vi "UHR-Fleezers Control (host) - 10.3.vi"() -> ()   [LabVIEW 2010] (continued)
            n263 = local write "Overflow (data lost)"(FALSE ("Overflow (data lost)")) -> ()
          }
        }
        n264 = case shown="False" w2065 {
          selector: w2065 -> [_ w2081]
          tunnel: w2064 -> [w2080 _]
          tunnel: [w2080 w2081] -> w2063
          frame False {
            n265 = property on="2D or 1D Scan" class="Bool (strict)"("Val(Sgnl)"=w2080) -> ()  [unwired: 2 in, 2 out]
            n266 = property on="Confocal Image" class="Bool (strict)"("Value"=FALSE ("Start Confocal Map")) -> ()  [unwired: 2 in, 2 out]
          }
          frame True {
          }
        }
        n267 = local write "MCL Scanning"(w2070) -> ()
        n268 = local read "AO1"() -> (w2067:dbl)
        n269 = local read "AO2"() -> (w2066:dbl)
        n270 = case shown="True" "Center Scan" {
          tunnel: w2075 -> [w2088 w2200]
          tunnel: w2074 -> [w2087 w2199]
          tunnel: [w2086 w2198] -> w2072
          tunnel: [w2085 w2197] -> w2071
          tunnel: [w2083 w2184] -> w2069
          tunnel: [w2082 w2183] -> w2068
          tunnel: w2067 -> [w2083 w2189]
          tunnel: w2066 -> [w2082 w2192]
          tunnel: w2063 -> [_ _]
          frame False {
            w2084 = TRUE ("AI to FIFO")
            n271 = xnode "Read/Write Control"("FPGA VI Reference In"=w2088, "error in"=w2087, "AI to FIFO"=w2084, "APD to FIFO"=w2084, "Start scan (MCL)"=w2084) -> ("FPGA VI Reference Out"=w2086:T19, "error out"=w2085:errorcluster)
          }
          frame True {
            w2196 = TRUE ("AI to FIFO")
            n272 = local read "Scan steps (MCL)"() -> (w2175:u64)
            n273 = local read "Scan lines (y)"() -> (w2171:u64)
            n274 = local read "Fast Scan Dir"() -> (w2182:bool)
            n275 = local read "Actual MCL Inc (V)"() -> (w2172:dbl)
            n276 = Decrement(x=w2171) -> (x-1=w2170:u64)
            n277 = Decrement(x=w2175) -> (x-1=w2174:u64)
            n278 = Multiply(x=w2172, y=w2170) -> (x*y=w2169:dbl)
            n279 = Divide(x=w2169, y=2.0) -> (x/y=w2179:dbl)
            n280 = Multiply(x=w2172, y=w2174) -> (x*y=w2173:dbl)
            n281 = Divide(x=w2173, y=2.0) -> (x/y=w2178:dbl)
            n282 = Select(t=w2178, s=w2182, f=w2179) -> (s? t:f=w2177:dbl)
            n283 = Select(t=w2179, s=w2182, f=w2178) -> (s? t:f=w2181:dbl)
            n284 = Subtract(x=w2189, y=w2181) -> (x-y=w2180:dbl)
            n285 = Subtract(x=w2192, y=w2177) -> (x-y=w2176:dbl)
            n286 = local read "2D or 1D Scan"() -> (w2194:bool)
            n287 = Not(x=w2182) -> (.not. x?=w2188:bool)
            n288 = Not(x=w2194) -> (.not. x?=w2190:bool)
            n289 = And(x=w2182, y=w2190) -> (x .and. y?=w2191:bool)
            n290 = And(x=w2190, y=w2188) -> (x .and. y?=w2193:bool)
            n291 = Select(t=w2192, s=w2193, f=w2176) -> (s? t:f=w2183:dbl)
            n292 = Select(t=w2189, s=w2191, f=w2180) -> (s? t:f=w2184:dbl)
            n293 = call "Volt to I16.vi"("Voltage In"=w2184) -> ("I16 Voltage Out"=w2187:i16)
            n294 = call "Volt to I16.vi"("Voltage In"=w2183) -> ("I16 Voltage Out"=w2186:i16)
            n295 = xnode "Read/Write Control"("FPGA VI Reference In"=w2200, "error in"=w2199, "AI to FIFO"=w2196, "APD to FIFO"=w2196, "Start scan (MCL)"=w2196, "AO1"=w2187, "AO2"=w2186) -> ("FPGA VI Reference Out"=w2198:T19, "error out"=w2197:errorcluster)
          }
        }
        "Initial Y" <- w2069
        "Initial X" <- w2068
        "wait to reset values" <- w2070
      }
    }
    n296 = local read "Trap Pos Elements/DMA read"() -> (w1019:u32)
    n297 = local read "Trap AI Elements/DMA read"() -> (w1104:u32)
    n298 = local read "APD Elements/DMA read"() -> (w1064:u32)
    n299 = xnode "Get APD Data"("FPGA VI Reference In"=w1023, "error in"=w1022, "Number of Elements"=w1064, "Timeout (ms)"=-1) -> ("Data"=w1063:u32[], "Elements Remaining"=→"APD FIFO Elements Remaining":u32)  [unwired: 2 out]
    n300 = xnode "Invoke Method"("FPGA VI Reference In"=w1023, "error in"=w1022, "Number of Elements"=w1019, "Timeout (ms)"=-1) -> ("Data"=w982:u16[], "Elements Remaining"=→"Trap Pos FIFO El Remaining":u32)  [unwired: 2 out]
    n301 = xnode "Get Trap Data"("FPGA VI Reference In"=w1023, "error in"=w1022, "Number of Elements"=w1104, "Timeout (ms)"=-1 ("Timeout")) -> ("FPGA VI Reference Out"=w1093:T19, "error out"=w1092:errorcluster, "Data"=w983:i16[], "Elements Remaining"=w1239:u32)
    "FIFO El. Rem." <- w1239
    n302 = local read "Trap AI FIFO Depth"() -> (w1241:u32)
    n303 = Subtract(x=w1241, y=w1104) -> (x-y=w1240:u32)
    n304 = Decimate 1D Array(w982) -> (w979:u16[], w981:u16[], w980:u16[])
    n305 = Divide(x=w1239, y=w1240) -> (x/y=w1238:dbl)
    "Buffer Status" <- w1238
    n306 = To Unsigned Long Integer(number=w979) -> (unsigned 32bit integer=w978:u32[])
    n307 = Join Numbers(hi=w981, lo=w980) -> ((hi.lo)=w977:u32[])
    n308 = Equal?(x=w1238, y=1.0) -> (x = y?=w1236:bool)
    n309 = Join Numbers(hi=w978, lo=w977) -> ((hi.lo)=w971:u64[])
    n310 = call "IR AOM word to freq - vec.vi"("Frequency Word In (double vec)"=w971) -> ("Frequency Out"=w1018:dbl[])
    n311 = case "Alert buffer overflow" shown="True" w1236 {
      frame False {
      }
      frame True {
        n312 = call <vilib>:"Beep.vi"() -> ()  [unwired: 3 in, 9 out]
        "Overflow (data lost)" <- TRUE ("Overflow (data lost)")
      }
    }
    n313 = Decimate 1D Array(w1018) -> (w1017:dbl[], w1016:dbl[])
    n314 = Build Array(w1017, w1016) -> (w1015:dbl[][])
    n315 = local read "Trap Sets"() -> (w1103:u32)
    n316 = case "Deinterlace trap data, average down PSD" shown="1, Default" w1103 {
      tunnel: w983 -> [w2357 w2422]
      tunnel: [w2354 w2419] -> w1096
      tunnel: [w2357 w2421] -> w974
      tunnel: "Detector Type" -> [w2356 w2417]
      tunnel: [w2355 w2420] -> w1095
      tunnel: [w2353 w2418] -> w1211
      frame 1, Default {
        n317 = Divide(x=w2357, y=3276.7) -> (x/y=w2358:dbl[])
        n318 = Decimate 1D Array(w2358) -> (w2367:dbl[], w2366:dbl[], w2365:dbl[], w2364:dbl[], w2363:dbl[], w2362:dbl[], w2361:dbl[], w2360:dbl[])
        n319 = case shown="\"IR-QPD + PSD + FB-QPD position\"" w2356 {
          tunnel: w2367 -> [w2391 w2416]
          tunnel: w2366 -> [w2390 w2415]
          tunnel: w2365 -> [w2375 w2393]
          tunnel: w2364 -> [w2376 w2403]
          tunnel: w2363 -> [w2389 w2414]
          tunnel: w2362 -> [w2388 w2413]
          tunnel: w2361 -> [w2372 w2394]
          tunnel: w2360 -> [w2371 w2392]
          tunnel: [w2370 w2400] -> w2355
          tunnel: [w2369 w2399] -> w2354
          tunnel: [w2368 w2398] -> w2353
          frame "IR-QPD + PSD + FB-QPD", Default {
            w2368 = 0  # Channel pattern
            n320 = Divide(x=w2391, y=w2376) -> (x/y=w2378:dbl[])
            n321 = Divide(x=w2390, y=w2376) -> (x/y=w2377:dbl[])
            n322 = Divide(x=w2389, y=w2372) -> (x/y=w2374:dbl[])
            n323 = Divide(x=w2388, y=w2371) -> (x/y=w2373:dbl[])
            n324 = Build Array(w2378, w2377, w2376, w2375, w2374, w2373, w2372, w2371) -> (w2369:dbl[][])
            n325 = Bundle("T1 Y", "T1 X", "T1 Sum", "FB Sum", "PSD Y", "PSD X", "PSD Y Sum", "PSD X Sum") -> (w2387:T35)  [unwired: 1 out]
            n326 = Cluster To Array(cluster=w2387) -> (array=w2370:string[])
          }
          frame "IR-QPD + PSD + FB-QPD position" {
            w2398 = 3  # Channel pattern
            n327 = Negate(x=w2394) -> (-x=w2395:dbl[])
            n328 = Divide(x=w2416, y=w2403) -> (x/y=w2405:dbl[])
            n329 = Divide(x=w2415, y=w2403) -> (x/y=w2404:dbl[])
            n330 = Divide(x=w2414, y=w2394) -> (x/y=w2402:dbl[])
            n331 = Divide(x=w2413, y=w2395) -> (x/y=w2401:dbl[])
            n332 = Build Array(w2405, w2404, w2403, w2392, w2393, w2402, w2401, w2394) -> (w2399:dbl[][])
            n333 = Bundle("T1 Y", "T1 X", "T1 Sum", "FB X", "FB Sum", "PSD Y", "PSD X", "PSD Y Sum") -> (w2412:T35)  [unwired: 1 out]
            n334 = Cluster To Array(cluster=w2412) -> (array=w2400:string[])
          }
        }
      }
      frame 2 {
        n335 = case shown="\"IR-QPD + PSD + FB-QPD X position\"" w2417 {
          tunnel: w2422 -> [w2484 w2551 w2622]
          tunnel: [w2423 w2542 w2553] -> w2421
          tunnel: [w2450 w2533 w2600] -> w2420
          tunnel: [w2449 w2496 w2567] -> w2419
          tunnel: [w2443 w2531 w2598] -> w2418
          frame "IR-QPD + PSD + FB-QPD", Default {
            w2443 = 1  # Channel pattern
            # "time average x2 the 4th signal and the 4 psd signals (detection laser)"
            # "deinterlace 3 signals from qpd"
            n336 = Decimate 1D Array(w2484) -> (w2483:i16[], w2482:i16[], w2448:i16[], w2481:i16[], w2471:i16[], w2469:i16[], w2468:i16[], w2466:i16[])
            n337 = Decimate 1D Array(w2448) -> (w2447:i16[], w2446:i16[])
            n338 = Decimate 1D Array(w2483) -> (w2480:i16[], w2452:i16[])
            n339 = Decimate 1D Array(w2482) -> (w2479:i16[], w2477:i16[])
            n340 = Decimate 1D Array(w2481) -> (w2478:i16[], w2476:i16[])
            n341 = call "downsample 1D array - double.vi"("Ave N"=2.0, "Array In"=w2471) -> ("Array Out"=w2470:dbl[])  [unwired: 1 out]
            n342 = call "downsample 1D array - double.vi"("Ave N"=2.0, "Array In"=w2469) -> ("Array Out"=w2451:dbl[])  [unwired: 1 out]
            n343 = call "downsample 1D array - double.vi"("Ave N"=2.0, "Array In"=w2468) -> ("Array Out"=w2467:dbl[])  [unwired: 1 out]
            n344 = call "downsample 1D array - double.vi"("Ave N"=2.0, "Array In"=w2466) -> ("Array Out"=w2465:dbl[])  [unwired: 1 out]
            n345 = Interleave 1D Arrays(w2480, w2479, w2478, w2452, w2477, w2476, w2447, w2446, w2470, w2451, w2467, w2465) -> (w2464:dbl[])
            n346 = Divide(x=w2464, y=3276.7) -> (x/y=w2463:dbl[])
            n347 = Decimate 1D Array(w2463) -> (w2462:dbl[], w2461:dbl[], w2460:dbl[], w2459:dbl[], w2458:dbl[], w2457:dbl[], w2445:dbl[], w2444:dbl[], w2456:dbl[], w2455:dbl[], w2454:dbl[], w2453:dbl[])
            n348 = Divide(x=w2462, y=w2460) -> (x/y=w2430:dbl[])
            n349 = Divide(x=w2461, y=w2460) -> (x/y=w2429:dbl[])
            n350 = Divide(x=w2459, y=w2457) -> (x/y=w2428:dbl[])
            n351 = Divide(x=w2458, y=w2457) -> (x/y=w2427:dbl[])
            n352 = Divide(x=w2456, y=w2454) -> (x/y=w2426:dbl[])
            n353 = Divide(x=w2455, y=w2453) -> (x/y=w2425:dbl[])
            n354 = Build Array(w2430, w2429, w2460, w2428, w2427, w2457, w2445, w2444, w2426, w2425, w2454, w2453) -> (w2449:dbl[][])
            n355 = Bundle("T1 Y", "T1 X", "T1 Sum", "T2 Y", "T2 X", "T2 Sum", "T1 FB Sum", "T2 FB Sum", "PSD Y", "PSD X", "PSD Y Sum", "PSD X Sum") -> (w2431:T36)  [unwired: 1 out]
            n356 = To Word Integer(number=w2464) -> (16bit integer=w2423:i16[])
            n357 = Cluster To Array(cluster=w2431) -> (array=w2450:string[])
          }
          frame "IR-QPD + PSD + FB-QPD X position" {
            w2531 = 2  # Channel pattern
            # "time average x2 the 3 psd signals (detection laser)"
            # "deinterlace 3 signals from qpds"
            n358 = Decimate 1D Array(w2551) -> (w2550:i16[], w2549:i16[], w2532:i16[], w2548:i16[], w2494:i16[], w2491:i16[], w2488:i16[], w2519:i16[])
            n359 = Decimate 1D Array(w2532) -> (w2517:i16[], w2515:i16[])
            n360 = Decimate 1D Array(w2550) -> (w2547:i16[], w2534:i16[])
            n361 = Decimate 1D Array(w2549) -> (w2546:i16[], w2544:i16[])
            n362 = Decimate 1D Array(w2548) -> (w2545:i16[], w2543:i16[])
            n363 = Decimate 1D Array(w2519) -> (w2518:i16[], w2516:i16[])
            n364 = call "downsample 1D array - I16.vi"("Ave N"=2.0, "Array In"=w2494) -> ("Array Out"=w2492:i16[])  [unwired: 1 in]
            n365 = call "downsample 1D array - I16.vi"("Ave N"=2.0, "Array In"=w2488) -> ("Array Out"=w2486:i16[])  [unwired: 1 in]
            n366 = call "downsample 1D array - I16.vi"("Ave N"=2.0, "Array In"=w2491) -> ("Array Out"=w2489:i16[])  [unwired: 1 in]
            n367 = Interleave 1D Arrays(w2547, w2546, w2545, w2534, w2544, w2543, w2518, w2517, w2516, w2515, w2492, w2489, w2486) -> (w2542:i16[])
            n368 = Divide(x=w2542, y=3276.7) -> (x/y=w2541:dbl[])
            n369 = Decimate 1D Array(w2541) -> (w2540:dbl[], w2539:dbl[], w2538:dbl[], w2537:dbl[], w2536:dbl[], w2535:dbl[], w2507:dbl[], w2505:dbl[], w2504:dbl[], w2502:dbl[], w2501:dbl[], w2500:dbl[], w2497:dbl[])
            n370 = Negate(x=w2497) -> (-x=w2495:dbl[])
            n371 = Divide(x=w2501, y=w2497) -> (x/y=w2499:dbl[])
            n372 = Divide(x=w2500, y=w2495) -> (x/y=w2498:dbl[])
            n373 = Divide(x=w2540, y=w2538) -> (x/y=w2523:dbl[])
            n374 = Divide(x=w2539, y=w2538) -> (x/y=w2522:dbl[])
            n375 = Divide(x=w2537, y=w2535) -> (x/y=w2521:dbl[])
            n376 = Divide(x=w2536, y=w2535) -> (x/y=w2520:dbl[])
            n377 = Divide(x=w2507, y=w2505) -> (x/y=w2506:dbl[])
            n378 = Divide(x=w2504, y=w2502) -> (x/y=w2503:dbl[])
            n379 = Build Array(w2523, w2522, w2538, w2521, w2520, w2535, w2506, w2505, w2503, w2502, w2499, w2498, w2497) -> (w2496:dbl[][])
            n380 = Bundle("T1 Y", "T1 X", "T1 Sum", "T2 Y", "T2 X", "T2 Sum", "T1 FB X", "T1 FB Sum", "T2 FB X", "T2 FB Sum", "PSD Y", "PSD X", "PSD Y Sum") -> (w2524:T37)  [unwired: 1 out]
            n381 = Cluster To Array(cluster=w2524) -> (array=w2533:string[])
          }
          frame "IR-QPD + PSD + FB-QPD XY positions" {
            w2598 = 4  # Channel pattern
            # "time average x2 the 3 psd signals (detection laser)"
            # "deinterlace 3 signals from qpds"
            n382 = Decimate 1D Array(w2622) -> (w2621:i16[], w2620:i16[], w2599:i16[], w2619:i16[], w2565:i16[], w2611:i16[], w2610:i16[], w2587:i16[])
            n383 = Decimate 1D Array "Feedback Sum"(w2599) -> (w2583:i16[], w2581:i16[])
            n384 = Decimate 1D Array "QPD Y"(w2621) -> (w2618:i16[], w2601:i16[])
            n385 = Decimate 1D Array "QPD X"(w2620) -> (w2617:i16[], w2615:i16[])
            n386 = Decimate 1D Array "Feedback Y"(w2565) -> (w2564:i16[], w2563:i16[])
            n387 = Decimate 1D Array "QPD Sum"(w2619) -> (w2616:i16[], w2614:i16[])
            n388 = Decimate 1D Array "Feedback X"(w2587) -> (w2584:i16[], w2582:i16[])
            n389 = call "downsample 1D array - double.vi"("Ave N"=2.0, "Array In"=w2611) -> ("Array Out"=w2586:dbl[])  [unwired: 1 out]
            n390 = call "downsample 1D array - double.vi"("Ave N"=2.0, "Array In"=w2610) -> ("Array Out"=w2585:dbl[])  [unwired: 1 out]
            n391 = Interleave 1D Arrays(w2618, w2617, w2616, w2601, w2615, w2614, w2564, w2584, w2583, w2563, w2582, w2581, w2586, w2585) -> (w2609:dbl[])
            n392 = Divide(x=w2609, y=3276.7) -> (x/y=w2608:dbl[])
            n393 = Decimate 1D Array(w2608) -> (w2607:dbl[], w2606:dbl[], w2605:dbl[], w2604:dbl[], w2603:dbl[], w2602:dbl[], w2560:dbl[], w2574:dbl[], w2558:dbl[], w2559:dbl[], w2572:dbl[], w2556:dbl[], w2570:dbl[], w2568:dbl[])
            n394 = Negate(x=w2568) -> (-x=w2566:dbl[])
            n395 = Divide(x=w2570, y=w2566) -> (x/y=w2569:dbl[])
            n396 = Divide(x=w2559, y=w2556) -> (x/y=w2555:dbl[])
            n397 = Divide(x=w2560, y=w2558) -> (x/y=w2557:dbl[])
            n398 = Divide(x=w2607, y=w2605) -> (x/y=w2591:dbl[])
            n399 = Divide(x=w2606, y=w2605) -> (x/y=w2590:dbl[])
            n400 = Divide(x=w2604, y=w2602) -> (x/y=w2589:dbl[])
            n401 = Divide(x=w2603, y=w2602) -> (x/y=w2588:dbl[])
            n402 = Divide(x=w2574, y=w2558) -> (x/y=w2573:dbl[])
            n403 = Divide(x=w2572, y=w2556) -> (x/y=w2571:dbl[])
            n404 = Build Array(w2591, w2590, w2605, w2589, w2588, w2602, w2557, w2573, w2558, w2555, w2571, w2556, w2569, w2568) -> (w2567:dbl[][])
            n405 = Bundle("T1 Y", "T1 X", "T1 Sum", "T2 Y", "T2 X", "T2 Sum", "T1 FB Y", "T1 FB X", "T1 FB Sum", "T2 FB Y", "T2 FB X", "T2 FB Sum", "PSD X", "PSD Y Sum") -> (w2554:T38)  [unwired: 1 out]
            n406 = To Word Integer(number=w2609) -> (16bit integer=w2553:i16[])
            n407 = Cluster To Array(cluster=w2554) -> (array=w2600:string[])
          }
        }
      }
    }
    "AI labels" <- w1095
    n408 = Decimate 1D Array(w1063) -> (w1091:u32[], w1027:u32[])
    n409 = local read "DMA Update Period (s)"() -> (w1105:dbl)
    n410 = local read "BD 1 Frequency 2 (MHz)"() -> (w966:dbl)
    n411 = local read "BD 1 Frequency 1 (MHz)"() -> (w967:dbl)
    n412 = Build Array(w1091, w1027) -> (w1173:u32[][])
    n413 = local read "Data Period (s)"() -> (w1076:dbl)
    n414 = Decimate 1D Array(w974) -> (w998:i16[], w997:i16[], w995:i16[], w994:i16[])  [unwired: 9 out]
    n415 = To Double Precision Float(number=w1173) -> (double precision float=w1174:dbl[][])
    n416 = local read "APD Integration Time (s)"() -> (w1040:dbl)
    n417 = Divide(x=w998, y=w997) -> (x/y=w999:dbl[])
    n418 = Divide(x=w995, y=w994) -> (x/y=w996:dbl[])
    n419 = feedback #1(0.0) -> (w1012:dbl)
    n420 = Add(x=w1105, y=w1012) -> (x+y=w1213:dbl)
    n421 = feedback-in #1(w1213) -> ()
    n422 = local read "AOM X Cal (nm/MHz)"() -> (w964:dbl)
    n423 = To Time Stamp(1:w1012) -> (0:w1011:timestamp)
    n424 = Split 1D Array(array=w999, index="N El. to Ave.") -> (second subarray=w1002:dbl[])  [unwired: 1 out]
    n425 = Split 1D Array(array=w996, index="N El. to Ave.") -> (second subarray=w1001:dbl[])  [unwired: 1 out]
    n426 = local read "Trap X AI1 (DMA)"() -> (w1000:T13)
    n427 = Multiply(x=w1076, y="Trap Disp. Downsample") -> (x*y=w1013:dbl)
    "Display Period (s)" <- w1013
    n428 = Bundle("BD 1 Frequency 1 (MHz)"=w967, "BD 1 Frequency 2 (MHz)"=w966) -> (w968:T39)  [unwired: 1 out]
    n429 = for "Trap AI" {
      tunnel: [w2352] -> w1207 mode=indexing
      tunnel: w1011 -> [w2342]
      tunnel: "Trap Disp. Downsample" -> [w2350]
      tunnel: w1096 -> [w2348] mode=indexing
      tunnel: w1076 -> [w2347]
      tunnel: w1095 -> [w2346] mode=indexing
      tunnel: w1010 -> [w2345]
      tunnel: [w2344] -> w1051 mode=indexing
      tunnel: w1013 -> [w2343]
      workers-P: _ -> [_]
      n430 = Bundle By Name("Y"=w2348, "dt"=w2347) -> (w2349:waveform(dbl))  [unwired: 1 out]
      n431 = Set Waveform Attribute(5:w2346, 6:w2345, 7:w2349) -> (3:w2344:waveform(dbl))  [unwired: 1 in, 2 out]
      n432 = call "downsample 1D array - double.vi"("Ave N"=w2350, "Array In"=w2348) -> ("Array Out"=w2351:dbl[])  [unwired: 1 out]
      n433 = Bundle By Name(cluster=w2344, "t0"=w2342, "Y"=w2351, "dt"=w2343) -> (w2352:waveform(dbl))
    }
    n434 = call <vilib>:"Mean.vi"("X"=w1001) -> ("mean"=w989:dbl)  [unwired: 1 out]
    n435 = call <vilib>:"Mean.vi"("X"=w1002) -> ("mean"=w990:dbl)  [unwired: 1 out]
    n436 = Cluster To Array(cluster=w968) -> (array=w965:dbl[])
    n437 = Reciprocal(x=w1013) -> (1/x=→"Trap Disp. Freq. (Hz)":dbl)
    n438 = local read "Data points/scans (MCL)"() -> (w1185:dbl)
    n439 = To Fixed-Point(number=w989) -> (fixed-point=w987:fxp<+/-,16,1>)  [unwired: 1 in]
    n440 = To Fixed-Point(number=w990) -> (fixed-point=w988:fxp<+/-,16,1>)  [unwired: 1 in]
    n441 = Bundle("Trap 1 Pos.", "Trap 2 Pos.") -> (w1009:cluster{string, string})  [unwired: 1 out]
    n442 = Bundle By Name(cluster=w1000, "Set 1"=w988, "Set 2"=w987) -> (→"Trap X AI1 (DMA)":T13)
    n443 = Cluster To Array(cluster=w1009) -> (array=w1006:string[])
    n444 = for "Trap Position" {
      tunnel: w1015 -> [w1257] mode=indexing
      tunnel: "Trap Disp. Downsample" -> [w1256]
      tunnel: w1013 -> [w1254]
      tunnel: w1011 -> [w1253]
      tunnel: w1010 -> [w1251]
      tunnel: w1006 -> [w1250] mode=indexing
      tunnel: [w1249] -> w963 mode=indexing
      tunnel: w965 -> [w1247] mode=indexing
      tunnel: w964 -> [w1245]
      n445 = call "downsample 1D array - double.vi"("Ave N"=w1256, "Array In"=w1257) -> ("Array Out"=w1255:dbl[])  [unwired: 1 out]
      n446 = Subtract(x=w1255, y=w1247) -> (x-y=w1248:dbl[])
      n447 = Multiply(x=w1245, y=w1248) -> (x*y=w1246:dbl[])
      n448 = Bundle By Name("Y"=w1246, "dt"=w1254, "t0"=w1253) -> (w1252:waveform(dbl))  [unwired: 1 out]
      n449 = Set Waveform Attribute(5:w1250, 6:w1251, 7:w1252) -> (3:w1249:waveform(dbl))  [unwired: 1 in, 2 out]
    }
    "Trap Positions" <- w963
    n450 = Bundle("APD 1", "APD 2") -> (w1206:cluster{string, string})  [unwired: 1 out]
    n451 = Cluster To Array(cluster=w1206) -> (array=w1203:string[])
    n452 = for "APD" {
      tunnel: w1174 -> [w2331] mode=indexing
      tunnel: w1040 -> [w2339]
      tunnel: [w2335] -> w1047 mode=indexing
      tunnel: "APD Disp. Scale" -> [w2336]
      tunnel: w1010 -> [w2334]
      tunnel: w1203 -> [w2333] mode=indexing
      tunnel: "APD Disp. Downsample" -> [w2329]
      tunnel: [w2332] -> w1202
      workers-P: _ -> [_]
      tunnel: w1011 -> [w2328]
      n453 = call "integrate 1D array interval - double.vi"("Ave N"=w2329, "Array In"=w2331) -> ("Array Out"=w2330:dbl[])  [unwired: 1 out]
      n454 = Multiply(x=w2339, y=w2329) -> (x*y=w2332:dbl)
      n455 = Divide(x=w2330, y=w2336) -> (x/y=w2337:dbl[])
      n456 = Bundle By Name("t0"=w2328, "Y"=w2337, "dt"=w2332) -> (w2338:waveform(dbl))  [unwired: 1 out]
      n457 = Set Waveform Attribute(5:w2333, 6:w2334, 7:w2338) -> (3:w2335:waveform(dbl))  [unwired: 1 in, 2 out]
    }
    "APD Display Period (s)" <- w1202
    n458 = Reciprocal(x=w1202) -> (1/x=→"APD Display Freq. (Hz)":dbl)
    n459 = local read "Display Period (s)"() -> (w1075:dbl)
    n460 = Increment(x=w1185) -> (x+1=w1186:dbl)
    n461 = Index Array(array=w963, index=0) -> (element=w961:waveform(dbl))
    n462 = To Double Precision Float(number=w1091) -> (double precision float=w1090:dbl[])
    n463 = feedback #2(w1186) -> (w1189:dbl)
    n464 = Select(t=0, s=w1176, f=w1189) -> (s? t:f=w1182:dbl)
    n465 = Array Size(array=w1090) -> (size(s)=w1188:i32)
    n466 = Add(x=w1188, y=w1182) -> (x+y=w1183:dbl)
    n467 = Unbundle By Name(w961) -> ("Y"=w959:dbl[])
    n468 = feedback #3(w1091) -> (w1172:u32[])
    n469 = Build Array (concatenate)(w1172, w1091) -> (w1169:u32[])
    n470 = feedback #4(w1027) -> (w1046:u32[])
    n471 = Divide(x="Bead Sep. Int. Time (s)", y=w1075) -> (x/y=w957:dbl)
    n472 = Build Array (concatenate)(w1046, w1027) -> (w1045:u32[])
    n473 = Greater?(x=w1183, y=w1185) -> (0:w1184:bool)
    n474 = feedback #5(w959) -> (w960:dbl[])
    n475 = Build Array (concatenate)(w959, w960) -> (w958:dbl[])
    n476 = Select(t=w1182, s=w1184, f=w1183) -> (s? t:f=w1181:dbl)
    n477 = feedback-in #2(w1181) -> ()
    n478 = Array Size(array=w1169) -> (size(s)=w1166:i32)
    n479 = Array Size(array=w1091) -> (size(s)=w1168:i32)
    n480 = local read "MCL Scanning"() -> (w1179:bool)
    n481 = local read "APD Integration Time (s)"() -> (w1054:dbl)
    n482 = Build Array (concatenate)(w1047, w1207) -> (w1049:waveform(dbl)[])
    "All Signals" <- w1049
    n483 = Split 1D Array(array=w958, index=w957) -> (first subarray=w951:dbl[])  [unwired: 1 out]
    n484 = feedback-in #5(w951) -> ()
    n485 = Multiply(x=w1168, y="APD Ave N") -> (x*y=w1167:dbl)
    n486 = Greater?(x=w1166, y=w1167) -> (0:w1170:bool)
    n487 = Not(x=w1184) -> (.not. x?=w1178:bool)
    n488 = To Double Precision Float(number=w1027) -> (double precision float=w1026:dbl[])
    n489 = call <vilib>:"Mean.vi"("X"=w951) -> ("mean"=w950:dbl)  [unwired: 1 out]
    "Mean T1 Position (nm)" <- w950
    n490 = Subtract(x=w951, y=w950) -> (x-y=w956:dbl[])
    n491 = Square(x=w956) -> (x^2=w955:dbl[])
    n492 = And(x=w1178, y=w1179) -> (x .and. y?=w1180:bool)
    n493 = call <vilib>:"Mean.vi"("X"=w955) -> ("mean"=w954:dbl)  [unwired: 1 out]
    n494 = case shown="True" w1170 {
      tunnel: w1169 -> [w1912 w1919]
      tunnel: [w1912 w1917] -> w1110
      tunnel: w1167 -> [_ w1914]
      tunnel: w1166 -> [_ w1918]
      tunnel: w1045 -> [w1911 w1916]
      tunnel: [w1911 w1913] -> w1042
      frame False {
      }
      frame True {
        n495 = Subtract(x=w1918, y=w1914) -> (x-y=w1915:dbl)
        n496 = Array Subset(array=w1919, index=w1915, length=w1914) -> (w1917:u32[])
        n497 = Array Subset(array=w1916, index=w1915, length=w1914) -> (w1913:u32[])
      }
    }
    n498 = feedback-in #3(w1110) -> ()
    n499 = feedback-in #4(w1042) -> ()
    n500 = Or(x=w1180, y=w1176) -> (x .or. y?=w1177:bool)
    n501 = Square Root(x=w954) -> (sqrt(x)=w953:dbl)
    n502 = Equal?(x="Tab Control 6", y=T26."High Res Display") -> (x = y?=w1099:bool)
    n503 = Multiply(x="APD Disp. Scale", y=w1047) -> (x*y=w1056:waveform(dbl)[])
    n504 = Multiply(x="APD Disp. Downsample", y=w1054) -> (x*y=w1052:dbl)
    n505 = Multiply(x=10.0, y=w953) -> (x*y=→"Trap 1 Position RMS (A)":dbl)
    n506 = Divide(x=w1056, y=w1052) -> (x/y=w1024:waveform(dbl)[])
    n507 = Index Array(array=w1024, index=0) -> (element=w1034:waveform(dbl))
    n508 = case "For computing FFTs for display" shown="True" "Compute FFT" {
      tunnel: w1051 -> [_ w3175]
      frame False {
      }
      frame True {
        n509 = Build Array("FFT 1 Choice 1", "FFT 1 Choice 2", "FFT 2 Choice 1", "FFT 2 Choice 2") -> (w3168:u16[])
        n510 = Array Size(array=w3175) -> (size(s)=w3174:i32)
        n511 = feedback-in #6(w3168) -> ()
        n512 = feedback #6(u16[] [100, 100, 100, 100]) -> (w3169:u16[])
        n513 = feedback-in #7("# Spectra to Ave.") -> ()
        n514 = feedback #7("# Spectra to Ave.") -> (w3166:dbl)
        n515 = Not Equal?(x="# Spectra to Ave.", y=w3166) -> (x != y?=w3165:bool)
        n516 = Not Equal?(x=w3168, y=w3169) -> (x != y?=w3167:bool)
        n517 = feedback #8(1.0) -> (w3152:dbl)
        n518 = Compound Arithmetic op=OR("Reset FFT", w3167, w3165) -> (w3150:bool)
        n519 = Select(t=1.0, s=w3150, f=w3152) -> (s? t:f=w3154:dbl)
        n520 = Greater?(x=w3154, y="# Spectra to Ave.") -> (0:w3173:bool)
        n521 = Increment(x=w3154) -> (x+1=w3153:dbl)
        n522 = feedback-in #8(w3153) -> ()
        n523 = local read "DMA Update Period (s)"() -> (w3148:dbl)
        n524 = Multiply(x="# Spectra to Ave.", y=w3148) -> (x*y=→"Ave. Time (s)":dbl)
        n525 = Build Array(cluster{"f0":dbl, "df":dbl, "magnitude":dbl[]} {"f0"=0.0, "df"=0.0, "magnitude"=[]} ("PSD")) -> (w3157:cluster{"f0":dbl, "df":dbl, "magnitude":dbl[]}[])
        n526 = Build Array(w3157, w3157, w3157, w3157) -> (w3159:T40)
        n527 = feedback #9(w3159) -> (w3164:T40)
        n528 = for {
          N: 4 -> [_]
          tunnel: w3168 -> [w3197] mode=indexing
          tunnel: w3175 -> [w3198]
          tunnel: w3174 -> [w3200]
          tunnel: w3150 -> [w3193]
          tunnel: w3173 -> [w3192]
          tunnel: "# Spectra to Ave." -> [w3191]
          tunnel: [w3190] -> w3163 mode=indexing
          tunnel: w3164 -> [w3195] mode=indexing
          tunnel: [w3194] -> w3151 mode=indexing
          tunnel: w3154 -> [w3189]
          n529 = Less?(x=w3197, y=w3200) -> (x < y?=w3199:bool)
          n530 = Index Array(array=w3198, index=w3197) -> (element=w3196:waveform(dbl))
          n531 = case shown="True" w3199 {
            tunnel: w3196 -> [_ w3217]
            tunnel: w3195 -> [w3202 w3215]
            tunnel: [w3202 w3203] -> w3194
            tunnel: w3193 -> [_ w3214]
            tunnel: w3192 -> [_ w3207]
            tunnel: w3191 -> [_ w3206]
            tunnel: [cluster{"f0":dbl, "df":dbl, "magnitude":dbl[]} {"f0"=0.0, "df"=0.0, "magnitude"=[]} ("PSD") w3208] -> w3190
            tunnel: w3189 -> [_ w3205]
            frame False {
            }
            frame True {
              n532 = call <vilib>:"Std Deviation and Variance.vi"("X"=w3217) -> ("mean"=w3218:dbl)  [unwired: 1 in, 2 out]
              n533 = Subtract(x=w3217, y=w3218) -> (x-y=w3216:waveform(dbl))
              n534 = xnode "Spectral Measurements"("Signals"=w3216) -> ("PSD"=w3210:cluster{"f0":dbl, "df":dbl, "magnitude":dbl[]})  [unwired: 1 in, 1 out]
              n535 = case shown="False" w3214 {
                tunnel: w3215 -> [w3227 _]
                tunnel: [w3223 w3232] -> w3203
                tunnel: w3210 -> [w3226 w3233]
                tunnel: w3207 -> [w3225 _]
                frame False {
                  n536 = Build Array (concatenate)(w3227, w3226) -> (w3224:cluster{"f0":dbl, "df":dbl, "magnitude":dbl[]}[])
                  n537 = case shown="True" w3225 {
                    tunnel: w3224 -> [w3228 w3231]
                    tunnel: [w3228 w3229] -> w3223
                    frame False {
                    }
                    frame True {
                      n538 = Delete From Array(array=w3231, index=0) -> (array with subset deleted=w3229:cluster{"f0":dbl, "df":dbl, "magnitude":dbl[]}[])  [unwired: 1 in, 1 out]
                    }
                  }
                }
                frame True {
                  n539 = Build Array(w3233) -> (w3232:cluster{"f0":dbl, "df":dbl, "magnitude":dbl[]}[])
                }
              }
              n540 = for {
                tunnel: w3203 -> [w3222] mode=indexing
                tunnel: [w3221] -> w3213 mode=indexing
                workers-P: _ -> [_]
                n541 = Unbundle By Name(w3222) -> ("magnitude"=w3221:dbl[])
              }
              n542 = Transpose 2D Array(2D array=w3213) -> (transposed array=w3212:dbl[][])
              n543 = for {
                tunnel: w3212 -> [w3220] mode=indexing
                tunnel: [w3219] -> w3211 mode=indexing
                workers-P: _ -> [_]
                n544 = Add Array Elements(numeric array=w3220) -> (sum=w3219:dbl)
              }
              n545 = Select(t=w3206, s=w3207, f=w3205) -> (s? t:f=w3204:dbl)
              n546 = Divide(x=w3211, y=w3204) -> (x/y=w3209:dbl[])
              n547 = Bundle By Name(cluster=w3210, "magnitude"=w3209) -> (w3208:cluster{"f0":dbl, "df":dbl, "magnitude":dbl[]})
            }
          }
        }
        n548 = case shown="True" w3150 {
          tunnel: w3151 -> [w3182 w3188]
          tunnel: [w3182 w3183] -> w3149
          frame False {
          }
          frame True {
            n549 = Array Subset(array=w3188, index (row)=0 ("index"), length (row)=4 ("length"), index (col)=0 ("index"), length (col)=1 ("length")) -> (w3183:T40)
          }
        }
        n550 = feedback-in #9(w3149) -> ()
        n551 = Split 1D Array(array=w3163, index=2) -> (first subarray=→"FFT 1":cluster{"f0":dbl, "df":dbl, "magnitude":dbl[]}[], second subarray=→"FFT 2":cluster{"f0":dbl, "df":dbl, "magnitude":dbl[]}[])
      }
    }
    n552 = Index Array(array=w1024, index=1) -> (element=w1032:waveform(dbl))
    n553 = case "For displaying the high resolution display (no downsampling)" shown="True" w1099 {
      tunnel: w1051 -> [_ w1421]
      frame False {
      }
      frame True {
        n554 = Index Array(array=w1421, index="High Res. Display") -> (element=w1422:waveform(dbl))
        n555 = call <vilib>:"Std Deviation and Variance.vi"("X"=w1422) -> ("mean"=w1429:dbl, "standard deviation"=w1434:dbl)  [unwired: 1 in, 1 out]
        "Mean Intensity" <- w1429
        "Sigma" <- w1434
        n556 = Subtract(x=w1422, y=w1429) -> (x-y=w1428:waveform(dbl))
        n557 = Select(t=w1428, s="Subtract mean", f=w1422) -> (s? t:f=→"1 Channel":waveform(dbl))
        n558 = Divide(x=w1434, y=w1429) -> (x/y=→"Sigma/Mean":dbl)
        n559 = feedback #10(1) -> (w1423:i32)
        n560 = Greater Or Equal?(x=w1423, y="Slow mean N ave.") -> (x >= y?=w1436:bool)
        n561 = Increment(x=w1423) -> (x+1=w1438:i32)
        n562 = Select(t=1, s=w1436, f=w1438) -> (s? t:f=w1425:i32)
        n563 = feedback-in #10(w1425) -> ()
        n564 = feedback #11() -> (w1426:waveform(dbl))  [unwired: 1 out]
        n565 = case shown="Default" w1423 {
          tunnel: [w1441 w1444] -> w1427
          tunnel: w1426 -> [w1443 _]
          tunnel: w1422 -> [w1442 w1444]
          frame Default {
            n566 = call-poly <vilib>:"Append Waveforms.vi"("waveform B"=w1442, "waveform A"=w1443) -> ("waveform out"=w1441:waveform(dbl))  [unwired: 1 in, 8 out]
          }
          frame 1 {
          }
        }
        n567 = feedback-in #11(w1427) -> ()
        n568 = case shown="True" w1436 {
          tunnel: w1427 -> [_ w1440]
          frame False {
          }
          frame True {
            n569 = call <vilib>:"Mean.vi"("X"=w1440) -> ("mean"=→"Slow mean":dbl)  [unwired: 1 out]
          }
        }
      }
    }
    n570 = case "For plotting results of scanning MCL" shown="True" w1177 {
      tunnel: w1176 -> [_ w1952]
      tunnel: w1090 -> [_ w2048]
      tunnel: w1185 -> [_ _]
      tunnel: w1051 -> [_ w2022]
      tunnel: w1026 -> [_ w1953]
      tunnel: w1025 -> [_ w1926]
      frame False {
      }
      frame True {
        w1933 = u32 0 items=["Horizontal", "Vertical", "Central", "1st Diagonal", "2nd Diagonal"] ("Type of Symmetry")
        w1961 = u32 0 items=["Horizontal", "Vertical", "Central", "1st Diagonal", "2nd Diagonal"] ("Type of Symmetry")
        w1964 = u32 0 items=["Horizontal", "Vertical", "Central", "1st Diagonal", "2nd Diagonal"] ("Type of Symmetry")
        w1993 = u32 0 items=["Horizontal", "Vertical", "Central", "1st Diagonal", "2nd Diagonal"] ("Type of Symmetry")
        n571 = Index Array(array=w2022, index=10) -> (element=w2028:waveform(dbl))
        n572 = Index Array(array=w2022, index=11) -> (element=w2025:waveform(dbl))
        n573 = local read "Cycles/step (MCL)"() -> (w1978:u64)
        n574 = Index Array(array=w2022, index="Channel") -> (element=w2024:waveform(dbl))
        n575 = Unbundle(w1926) -> ("New Image"=w1925:T2, "New Image"=w1924:T2, "New Image"=w1923:T2, "New Image"=w1922:T2)
        n576 = Unbundle By Name(w2028) -> ("Y"=w1980:dbl[])
        n577 = Unbundle By Name(w2025) -> ("Y"=w1982:dbl[])
        n578 = Unbundle By Name(w2024) -> ("Y"=w1987:dbl[])
        n579 = call "downsample 1D array - double.vi"("Ave N"=w1978, "Array In"=w1980) -> ("Array Out"=w1979:dbl[])  [unwired: 1 out]
        n580 = call "downsample 1D array - double.vi"("Ave N"=w1978, "Array In"=w1982) -> ("Array Out"=w1981:dbl[])  [unwired: 1 out]
        n581 = call "downsample 1D array - double.vi"("Ave N"=w1978, "Array In"=w1987) -> ("Array Out"=w1986:dbl[])  [unwired: 1 out]
        n582 = feedback #12(w2048) -> (w2049:dbl[])
        n583 = Build Array (concatenate)(w2049, w2048) -> (w2030:dbl[])
        n584 = feedback #13(w1953) -> (w1955:dbl[])
        n585 = Build Array (concatenate)(w1955, w1953) -> (w1954:dbl[])
        n586 = local read "Scan steps (MCL)"() -> (w1935:u64)
        n587 = Select(t=w2048, s=w1952, f=w2030) -> (s? t:f=w2034:dbl[])
        n588 = feedback-in #12(w2034) -> ()
        n589 = Select(t=w1953, s=w1952, f=w1954) -> (s? t:f=w1936:dbl[])
        n590 = feedback-in #13(w1936) -> ()
        n591 = local read "Scan lines (y)"() -> (w1921:u64)
        n592 = local read "N APD Samp/step"() -> (w1937:dbl)
        n593 = feedback #14(w1979) -> (w2036:dbl[])
        n594 = Build Array (concatenate)(w2036, w1979) -> (w2027:dbl[])
        n595 = feedback #15(w1986) -> (w2046:dbl[])
        n596 = Build Array (concatenate)(w2046, w1986) -> (w2045:dbl[])
        n597 = feedback #16(w1981) -> (w2038:dbl[])
        n598 = Build Array (concatenate)(w2038, w1981) -> (w2039:dbl[])
        n599 = Select(t=w1979, s=w1952, f=w2027) -> (s? t:f=w1983:dbl[])
        n600 = feedback-in #14(w1983) -> ()
        n601 = Select(t=w1986, s=w1952, f=w2045) -> (s? t:f=w1985:dbl[])
        n602 = feedback-in #15(w1985) -> ()
        n603 = Select(t=w1981, s=w1952, f=w2039) -> (s? t:f=w1984:dbl[])
        n604 = feedback-in #16(w1984) -> ()
        n605 = Multiply(x=w1935, y=u64 2) -> (x*y=w1920:u64)
        n606 = call "integrate 1D array interval - double.vi"("Ave N"=w1937, "Array In"=w1936) -> ("Array Out"=w1948:dbl[])  [unwired: 1 out]
        n607 = call "integrate 1D array interval - double.vi"("Ave N"=w1937, "Array In"=w2034) -> ("Array Out"=w2033:dbl[])  [unwired: 1 out]
        n608 = Array Size(array=w1948) -> (size(s)=w1949:i32)
        n609 = Array Size(array=w2033) -> (size(s)=w2035:i32)
        n610 = Multiply(x=w1921, y=w1920) -> (x*y=w1951:u64)
        n611 = Multiply(x=w1921, y=w1920) -> (x*y=w2043:u64)
        n612 = call <vilib>:"Mean.vi"("X"=w1983) -> ("mean"=w1967:dbl)  [unwired: 1 out]
        n613 = Subtract(x=w1951, y=w1949) -> (x-y=w1942:u64)
        n614 = call <vilib>:"Mean.vi"("X"=w1985) -> ("mean"=w1972:dbl)  [unwired: 1 out]
        n615 = call <vilib>:"Mean.vi"("X"=w1984) -> ("mean"=w1970:dbl)  [unwired: 1 out]
        n616 = call <vilib>:"Mean.vi"("X"=w1948) -> ("mean"=w1939:dbl)  [unwired: 1 out]
        n617 = Subtract(x=w2043, y=w2035) -> (x-y=w1977:u64)
        n618 = call <vilib>:"Mean.vi"("X"=w2033) -> ("mean"=w1974:dbl)  [unwired: 1 out]
        n619 = Initialize Array(1.0 ("element"), w1942) -> (w1938:dbl[])
        n620 = Initialize Array(1.0 ("element"), w1977) -> (w1968:dbl[])
        n621 = Multiply(x=w1938, y=w1939) -> (x*y=w1940:dbl[])
        n622 = Multiply(x=w1968, y=w1970) -> (x*y=w1971:dbl[])
        n623 = Multiply(x=w1968, y=w1972) -> (x*y=w1973:dbl[])
        n624 = Multiply(x=w1968, y=w1967) -> (x*y=w1969:dbl[])
        n625 = Multiply(x=w1968, y=w1974) -> (x*y=w1975:dbl[])
        n626 = Build Array (concatenate)(w1983, w1969) -> (w2037:dbl[])
        n627 = Build Array (concatenate)(w1985, w1973) -> (w2041:dbl[])
        n628 = Build Array (concatenate)(w1984, w1971) -> (w2040:dbl[])
        n629 = Build Array (concatenate)(w1948, w1940) -> (w1950:dbl[])
        n630 = Build Array (concatenate)(w2033, w1975) -> (w2042:dbl[])
        n631 = Reshape Array(w2037, w1921, w1920) -> (w2003:dbl[][])
        n632 = Reshape Array(w1950, w1921, w1920) -> (w1946:dbl[][])
        n633 = Reshape Array(w2041, w1921, w1920) -> (w1995:dbl[][])
        n634 = Reshape Array(w2040, w1921, w1920) -> (w2010:dbl[][])
        n635 = Reshape Array(w2042, w1921, w1920) -> (w2020:dbl[][])
        n636 = Array Subset(array=w2010, index (col)=0 ("index"), length (col)=w1935) -> (w2015:dbl[][])  [unwired: 2 in]
        n637 = Array Subset(array=w2010, index (col)=w1935) -> (w2013:dbl[][])  [unwired: 3 in]
        n638 = Array Subset(array=w1995, index (col)=0 ("index"), length (col)=w1935) -> (w2001:dbl[][])  [unwired: 2 in]
        n639 = Array Subset(array=w1995, index (col)=w1935) -> (w1999:dbl[][])  [unwired: 3 in]
        n640 = Array Subset(array=w1946, index (col)=0 ("index"), length (col)=w1935) -> (w1945:dbl[][])  [unwired: 2 in]
        n641 = Array Subset(array=w1946, index (col)=w1935) -> (w1943:dbl[][])  [unwired: 3 in]
        n642 = Array Subset(array=w2020, index (col)=0 ("index"), length (col)=w1935) -> (w2019:dbl[][])  [unwired: 2 in]
        n643 = Array Subset(array=w2020, index (col)=w1935) -> (w2017:dbl[][])  [unwired: 3 in]
        n644 = Array Subset(array=w2003, index (col)=0 ("index"), length (col)=w1935) -> (w2008:dbl[][])  [unwired: 2 in]
        n645 = Array Subset(array=w2003, index (col)=w1935) -> (w2006:dbl[][])  [unwired: 3 in]
        n646 = for {
          tunnel: w2015 -> [w2057] mode=indexing
          tunnel: [w2056] -> w2014 mode=indexing
          workers-P: _ -> [_]
          n647 = Reverse 1D Array(array=w2057) -> (reversed array=w2056:dbl[])
        }
        n648 = for {
          tunnel: w2001 -> [w2053] mode=indexing
          tunnel: [w2052] -> w2000 mode=indexing
          workers-P: _ -> [_]
          n649 = Reverse 1D Array(array=w2053) -> (reversed array=w2052:dbl[])
        }
        n650 = for {
          tunnel: w1945 -> [w2051] mode=indexing
          tunnel: [w2050] -> w1944 mode=indexing
          workers-P: _ -> [_]
          n651 = Reverse 1D Array(array=w2051) -> (reversed array=w2050:dbl[])
        }
        n652 = for {
          tunnel: w2019 -> [w2059] mode=indexing
          tunnel: [w2058] -> w2018 mode=indexing
          workers-P: _ -> [_]
          n653 = Reverse 1D Array(array=w2059) -> (reversed array=w2058:dbl[])
        }
        n654 = for {
          tunnel: w2008 -> [w2055] mode=indexing
          tunnel: [w2054] -> w2007 mode=indexing
          workers-P: _ -> [_]
          n655 = Reverse 1D Array(array=w2055) -> (reversed array=w2054:dbl[])
        }
        n656 = Index Array(array=w2020, index (row)=0) -> (element=→"Waveform Graph":dbl[])  [unwired: 1 in]
        n657 = Add(x=w2014, y=w2013) -> (x+y=w2012:dbl[][])
        n658 = Add(x=w2000, y=w1999) -> (x+y=w1998:dbl[][])
        n659 = Add(x=w1944, y=w1943) -> (x+y=w1928:dbl[][])
        n660 = Add(x=w2018, y=w2017) -> (x+y=w1992:dbl[][])
        n661 = Add(x=w2007, y=w2006) -> (x+y=w2005:dbl[][])
        n662 = Divide(x=w1998, y=2) -> (x/y=w1996:dbl[][])
        n663 = Divide(x=w2012, y=2) -> (x/y=w1957:dbl[][])
        n664 = Divide(x=w2005, y=2) -> (x/y=w1959:dbl[][])
        n665 = To Single Precision Float(number=w1992) -> (single precision float=w1991:sgl[][])
        n666 = Transpose 2D Array(2D array=w1996) -> (transposed array=→"Data map":dbl[][])
        n667 = To Single Precision Float(number=w1928) -> (single precision float=w1932:sgl[][])
        n668 = To Single Precision Float(number=w1957) -> (single precision float=w1963:sgl[][])
        n669 = To Single Precision Float(number=w1959) -> (single precision float=w1960:sgl[][])
        n670 = call "IMAQ ArrayToImage"("Image Pixels (Float)"=w1991, "Image"=w1925) -> ("Image Out"=w1994:T2)  [unwired: 8 in, 1 out]
        n671 = call "IMAQ ArrayToImage"("Image Pixels (Float)"=w1932, "Image"=w1924) -> ("Image Out"=w1934:T2)  [unwired: 8 in, 1 out]
        n672 = call "IMAQ ArrayToImage"("Image Pixels (Float)"=w1963, "Image"=w1923) -> ("Image Out"=w1965:T2)  [unwired: 8 in, 1 out]
        n673 = call "IMAQ ArrayToImage"("Image Pixels (Float)"=w1960, "Image"=w1922) -> ("Image Out"=w1962:T2)  [unwired: 8 in, 1 out]
        n674 = call "IMAQ Symmetry"("Type of Symmetry"=w1993, "Image Src"=w1994) -> ("Image Dst Out"=w1989:T2)  [unwired: 3 in, 1 out]
        n675 = call "IMAQ Symmetry"("Type of Symmetry"=w1933, "Image Src"=w1934) -> ("Image Dst Out"=w1930:T2)  [unwired: 3 in, 1 out]
        n676 = call "IMAQ Symmetry"("Type of Symmetry"=w1964, "Image Src"=w1965) -> ("Image Dst Out"=→"Detection Laser X":T2)  [unwired: 3 in, 1 out]
        n677 = call "IMAQ Symmetry"("Type of Symmetry"=w1961, "Image Src"=w1962) -> ("Image Dst Out"=→"Detection Laser Y":T2)  [unwired: 3 in, 1 out]
        n678 = call "IMAQ Set Simple Calibration"("Calibration Axis Info"=T27 {"Origin Pixel"={"X"=0.0, "Y"=0.0}, "Angle Relative to Horizontal (deg)"=0.0, "Axis Reference"=0}, "Grid Descriptor"=T28 {"X Step"=0.3, "Y Step"=0.3, "Unit"=enum."Undefined"}, "Image"=w1989) -> ("Calibrated Image"=→"APD 1":T2)  [unwired: 7 in, 1 out]
        n679 = call "IMAQ Set Simple Calibration"("Calibration Axis Info"=T27 {"Origin Pixel"={"X"=0.0, "Y"=0.0}, "Angle Relative to Horizontal (deg)"=0.0, "Axis Reference"=0}, "Grid Descriptor"=T28 {"X Step"=0.3, "Y Step"=0.3, "Unit"=enum."Undefined"}, "Image"=w1930) -> ("Calibrated Image"=→"APD 2":T2)  [unwired: 7 in, 1 out]
      }
    }
    n680 = Subtract(x=w1032, y="APD 2 Offset") -> (x-y=w1029:waveform(dbl))
    n681 = Subtract(x=w1034, y="APD 1 Offset") -> (x-y=w1030:waveform(dbl))
    n682 = Index Array(array=w1049, index=3) -> (element=w1121:waveform(dbl))
    n683 = Index Array(array=w1049, index=6) -> (element=w1118:waveform(dbl))
    n684 = Build Array(w1030, w1029) -> (→"APD Chart":waveform(dbl)[])
    n685 = Array Size(array=w1110) -> (size(s)=w1165:i32)
    n686 = call <vilib>:"Std Deviation and Variance.vi"("X"=w1042) -> ("standard deviation"=w1041:dbl)  [unwired: 1 in, 2 out]
    n687 = Add Array Elements(numeric array=w1042) -> (sum=w1044:u32)
    n688 = Add Array Elements(numeric array=w1110) -> (sum=w1175:u32)
    n689 = call <vilib>:"Std Deviation and Variance.vi"("X"=w1110) -> ("standard deviation"=w1109:dbl)  [unwired: 1 in, 2 out]
    n690 = Divide(x="T1 offset_x (mV)", y=1000.0) -> (x/y=w1122:dbl)
    n691 = Divide(x=w1041, y=w1040) -> (x/y=w1037:dbl)
    "Rate sigma (Hz) 2" <- w1037
    n692 = Multiply(x=w1040, y=w1165) -> (x*y=w1043:dbl)
    "Int. Time (s)" <- w1043
    n693 = Divide(x=w1044, y=w1043) -> (x/y=w1038:dbl)
    "APD 2 Rate (Hz)" <- w1038
    n694 = Divide(x=w1175, y=w1043) -> (x/y=w1107:dbl)
    "APD 1 Rate (Hz)" <- w1107
    n695 = Divide(x=w1109, y=w1040) -> (x/y=w1108:dbl)
    "Rate sigma (Hz)" <- w1108
    n696 = Divide(x=w1037, y=w1038) -> (x/y=→"Sigma/Mean 2":dbl)
    n697 = Divide(x=w1108, y=w1107) -> (x/y=→"Sigma/Mean":dbl)
    n698 = Divide(x="T2 offset_x (mV)", y=1000.0) -> (x/y=w1120:dbl)
    n699 = case shown="0, Default" "Calibration" {
      tunnel: "T1 alpha_x (nm/V)" -> [_ w1888 w1909]
      tunnel: "T1 kappa_x (pN/nm)" -> [_ _ w1899]
      tunnel: "T2 alpha_x (nm/V)" -> [_ w1887 w1907]
      tunnel: "T2 kappa_x (pN/nm)" -> [_ _ w1900]
      tunnel: w1121 -> [w1870 w1885 w1905]
      tunnel: w1118 -> [w1869 w1883 w1903]
      tunnel: [w1870 w1882 w1902] -> w1151
      tunnel: [w1869 w1881 w1901] -> w1150
      tunnel: ["T1 X (V)" ("Label.Text") "T1 X (nm)" ("Label.Text") "T1 X (pN)" ("Label.Text")] -> w1139
      tunnel: ["T2 X (V)" ("Label.Text") "T2 X (nm)" ("Label.Text") "T2 X (pN)" ("Label.Text")] -> w1138
      tunnel: ["Position (V)" ("Label.Text") "Position (nm)" ("Label.Text") "Force (pN)" ("Label.Text")] -> w1140
      tunnel: w1120 -> [_ w1873 w1892]
      tunnel: w1122 -> [_ w1876 w1894]
      tunnel: ["Mean (V)" ("Label.Text") "Mean (nm)" ("Label.Text") "Mean (pN)" ("Label.Text")] -> w1135
      tunnel: ["Difference (V)" ("Label.Text") "Difference (nm)" ("Label.Text") "Difference (pN)" ("Label.Text")] -> w1057
      frame 0, Default {
      }
      frame 1 {
        n700 = Unbundle By Name(w1885) -> ("Y"=w1889:dbl[])
        n701 = Unbundle By Name(w1883) -> ("Y"=w1874:dbl[])
        n702 = Subtract(x=w1889, y=w1876) -> (x-y=w1877:dbl[])
        n703 = Subtract(x=w1874, y=w1873) -> (x-y=w1875:dbl[])
        n704 = Multiply(x=w1875, y=w1887) -> (x*y=w1884:dbl[])
        n705 = Multiply(x=w1888, y=w1877) -> (x*y=w1886:dbl[])
        n706 = Bundle By Name(cluster=w1883, "Y"=w1884) -> (w1881:waveform(dbl))
        n707 = Bundle By Name(cluster=w1885, "Y"=w1886) -> (w1882:waveform(dbl))
      }
      frame 2 {
        n708 = Unbundle By Name(w1905) -> ("Y"=w1910:dbl[])
        n709 = Unbundle By Name(w1903) -> ("Y"=w1908:dbl[])
        n710 = Subtract(x=w1908, y=w1892) -> (x-y=w1893:dbl[])
        n711 = Subtract(x=w1910, y=w1894) -> (x-y=w1895:dbl[])
        n712 = Compound Arithmetic op=MULTIPLY(w1893, w1907, w1900) -> (w1904:dbl[])
        n713 = Compound Arithmetic op=MULTIPLY(w1899, w1909, w1895) -> (w1906:dbl[])
        n714 = Bundle By Name(cluster=w1903, "Y"=w1904) -> (w1901:waveform(dbl))
        n715 = Bundle By Name(cluster=w1905, "Y"=w1906) -> (w1902:waveform(dbl))
      }
    }
    n716 = feedback-in #17("Calibration") -> ()
    n717 = feedback #17(u16 1 ("Calibration")) -> (w1142:u16)
    n718 = Not Equal?(x=w1142, y="Calibration") -> (x != y?=w1097:bool)
    n719 = Unbundle By Name(w1121) -> ("Y"=w1124:dbl[])
    n720 = Unbundle By Name(w1118) -> ("Y"=w1127:dbl[])
    n721 = Subtract(x=w1124, y=w1122) -> (x-y=w1125:dbl[])
    n722 = Subtract(x=w1127, y=w1120) -> (x-y=w1126:dbl[])
    n723 = Multiply(x=w1126, y="T2 alpha_x (nm/V)") -> (x*y=w1117:dbl[])
    n724 = Multiply(x="T1 alpha_x (nm/V)", y=w1125) -> (x*y=w1116:dbl[])
    n725 = Multiply(x=w1150, y=-1.0) -> (x*y=w1129:waveform(dbl))
    n726 = case shown="True" "Read Lateness and Rel Phase" {
      tunnel: w1093 -> [w1445 w1467]
      tunnel: w1092 -> [w1446 w1466]
      tunnel: [w1445 w1465] -> w1113
      tunnel: [w1446 w1464] -> w1112
      frame False {
      }
      frame True {
        n727 = xnode "Read/Write Control"("FPGA VI Reference In"=w1467, "error in"=w1466) -> ("FPGA VI Reference Out"=w1465:T19, "error out"=w1464:errorcluster, "GI Relative phase"=→"GI relative phase":i16, "Relative phase"=→"Relative phase (AI1)":i16, "AI Late Counter"=→"Late Counter (AI1)":u16, "GI Late Counter"=→"GI Late Counter":u16, "MCL Late Counter"=→"MCL Late Counter":u16, "MCL Relative Phase"=→"Relative Phase (MCL)":i16, "APD Acq Relative Phase"=→"APD Acq Relative Phase":i16, "APD 1 Gate Relative Phase"=→"APD 1 Gate Relative Phase":i16, "APD 2 Gate Relative Phase"=→"APD 2 Gate Relative Phase":i16, "APD Acq Late Counter"=→"APD Acq Late Counter":u16, "APD 1 Gate Late Counter"=→"APD 1 Gate Late Counter":u16, "APD 2 Gate Late Counter"=→"APD 2 Gate Late Counter":u16, "Green FB Relative Phase"=→"Relative phase (Green FB)":i16, "GI Relative phase 2"=→"GI relative phase 2":i16, "GI Late Counter 2"=→"GI Late Counter 2":u16, "Trap Pos FIFO Timeout"=→"Trap Pos FIFO Timeout":u16, "Trap AI FIFO Timeout"=→"Trap AI FIFO Timeout":u16)
      }
    }
    n728 = Subtract(x=w1117, y=w1116) -> (x-y=w1115:dbl[])
    n729 = Unbundle By Name(w1150) -> ("Y"=w1082:dbl[])
    n730 = Unbundle By Name(w1151) -> ("Y"=w1083:dbl[])
    n731 = Build Array(w1151, w1129) -> (→"Force":waveform(dbl)[])
    n732 = Subtract(x=w1115, y="Offset (nm)") -> (x-y=w1080:dbl[])
    n733 = call <vilib>:"Mean.vi"("X"=w1082) -> ("mean"=w1061:dbl)  [unwired: 1 out]
    "T2 X" <- w1061
    n734 = Absolute Value(x=w1083) -> (abs(x)=w1084:dbl[])
    n735 = Absolute Value(x=w1082) -> (abs(x)=w1085:dbl[])
    n736 = call <vilib>:"Mean.vi"("X"=w1083) -> ("mean"=w1062:dbl)  [unwired: 1 out]
    "T1 X" <- w1062
    n737 = Add(x=w1084, y=w1085) -> (x+y=w1086:dbl[])
    n738 = Bundle By Name(cluster=w1121, "Y"=w1080) -> (w1048:waveform(dbl))
    "Bead Separation" <- w1048
    n739 = Divide(x=w1086, y=2.0) -> (x/y=→"Vec Mean of T1 T2":dbl[])
    n740 = case shown="True" w1097 {
      tunnel: w1140 -> [_ w1863]
      tunnel: w1139 -> [_ w1862]
      tunnel: w1138 -> [_ w1861]
      tunnel: w1135 -> [_ w1860]
      tunnel: w1057 -> [_ w1859]
      frame False {
      }
      frame True {
        n741 = property on="Force" class="WFChart (strict)"("YScale.NameLbl.Text"=w1863) -> ()  [unwired: 2 in, 2 out]
        n742 = property on="T2 X" class="DigNum (strict)"("Caption.Text"=w1861) -> ()  [unwired: 2 in, 2 out]
        n743 = property on="T1 X" class="DigNum (strict)"("Caption.Text"=w1862) -> ()  [unwired: 2 in, 2 out]